vi "Host_timing_study_FPGA_check.vi"() -> ()   [LabVIEW 2019]
uses:
  <vilib>/Analysis/7linalg.llb/Eigenvalue and Vectors Output Option.ctl
  <vilib>/FPGAPlugInAG/PXIe-7915/niLvFpga_Open_PXIe-7915.vi
  <vilib>/rvi/interface/common/dynamic/niFpgaDynamicAddResources.vi
  <vilib>/Utility/error.llb/Error Cluster From Error Code.vi
  <vilib>/rvi/errors/niLvFpgaAdjustHostInterfaceError.vi
  <vilib>/FPGAPlugInAG/Dynamic/niLvFpga_Run_Dynamic.vi
  <vilib>/Analysis/baseanly.llb/Real Inverse Matrix.vi
  <vilib>/Analysis/Matrix/Numeric/Multiply/Multiply - RM,RM.vi
  <vilib>/Analysis/Matrix/Numeric/Add/Add - RM,RM.vi
  <vilib>/Analysis/Matrix/Numeric/Conversions/Matrix To Array - RM.vi
  <vilib>/Analysis/7linalg.llb/Real Eigenvalues and Vectors.vi
  <vilib>/FPGAPlugInAG/Dynamic/niLvFpga_Close_Dynamic.vi
  <vilib>/rvi/interface/nirviOpenFPGA/nirviOpenFPGA.xnode
  FPGA Bitfiles/Cholesky_SGL_19_nodes.lvbitx
  <vilib>/rvi/interface/nirviMethod/nirviMethod.xnode
  <vilib>/rvi/interface/nirviCloseFPGA/nirviCloseFPGA.xnode
  <vilib>/Analysis/NI_AALPro.lvlib
  <vilib>/Analysis/NI_AALBase.lvlib
  <vilib>/Analysis/Matrix/NI_Matrix.lvlib
  <vilib>/FPGAPlugInAG/Dynamic/niLvFpga_WriteFifo_Dynamic.vi
  <vilib>/rvi/errors/niLvFpgaMergeErrorWithErrorCode.vi
  <vilib>/FPGAPlugInAG/Dynamic/niLvFpga_ReadFifo_Dynamic.vi
panel:
  out "total run time (ms) 3":dbl
  out "total run time (ms) 2":dbl
  in  "stop":bool
  out "Eigenvalues":cdb[](array[numeric])
  out "total run time (ms)":dbl
  out "Frequencies":dbl[](array[numeric])
  out "K input":dbl[][](array[numeric])
  out "M input":dbl[][](array[numeric])
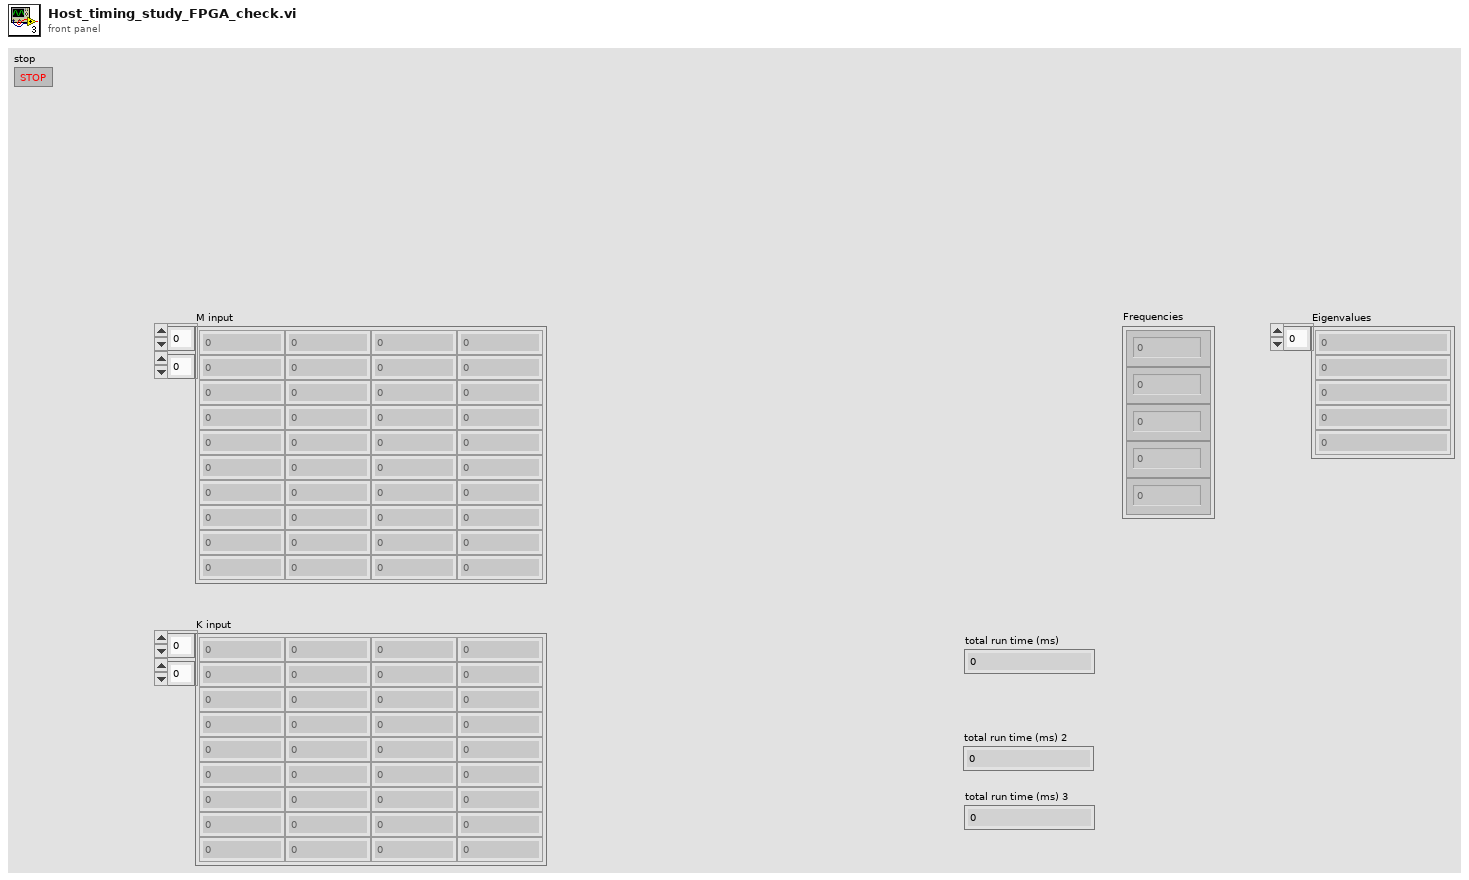
[diagram p1: front panel]
types:
  T1 = typedef "NI_AALPro.lvlib/Eigenvalue and Vectors Output Option.ctl" = i32
  T2 = typedef "NI_Matrix.lvlib/RealMatrix.ctl" = dbl[][]
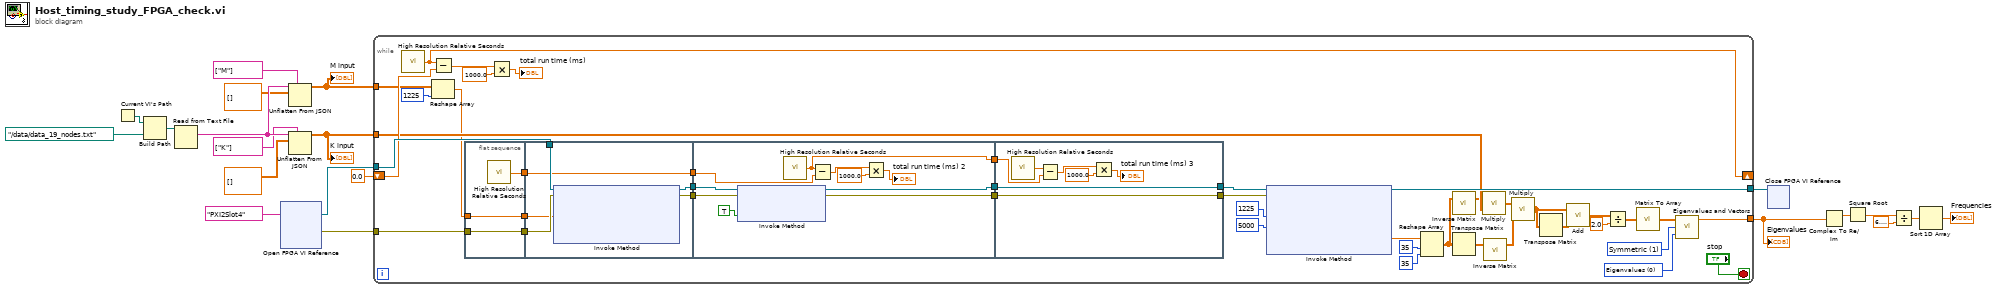
[diagram p0: block diagram]
diagram:
  n1 = Current VI's Path() -> (path=w15:path)
  n2 = Build Path(base path=w15, name or relative path=path "../data/data_19_nodes.txt") -> (appended path=w14:path)
  n3 = Read from Text File(file (use dialog)=w14) -> (text=w21:string)  [unwired: 3 in, 3 out]
  n4 = xnode "Open FPGA VI Reference"("resource name"=tag "PXI2Slot4") -> ("FPGA VI Reference Out"=w8:refnum<k20>, "error out"=w7:errorcluster)  [unwired: 1 in]
  n5 = Unflatten From JSON(path=string[] ["M"], JSON string=w21, type and defaults=dbl[][] []) -> (value=w3:dbl[][])  [unwired: 4 in, 1 out]
  "M input" <- w3
  n6 = Unflatten From JSON(path=string[] ["K"], JSON string=w21, type and defaults=dbl[][] []) -> (value=w4:dbl[][])  [unwired: 4 in, 1 out]
  "K input" <- w4
  n7 = while {
    tunnel: w8 -> [w64]
    tunnel: w7 -> [w63]
    tunnel: [w59] -> w5
    tunnel: w4 -> [w51]
    tunnel: w3 -> [w50]
    tunnel: [w57] -> w2
    shift-right: [w56] -> _
    shift-left: 0.0 ("relative seconds") -> [w55]
    stop <- "stop" stop-if-true
    w60 = T1 0 items=["Eigenvalues", "Eigenvalues & Vectors"] ("output option")
    w61 = 1 items=["General", "Symmetric"] ("matrix type")
    n8 = call <vilib>:"High Resolution Relative Seconds.vi"() -> ("relative seconds"=w56:dbl)
    n9 = Subtract(x=w56, y=w55) -> (x-y=w52:dbl)
    n10 = Reshape Array(w50, 1225 ("dimension size")) -> (w49:dbl[])
    n11 = flat-sequence {
      tunnel: w49 -> [w66]
      tunnel: w63 -> [w67]
      tunnel: [w67] -> w32
      tunnel: [w66] -> w31
      tunnel: [w65] -> w28
      tunnel: w64 -> [w73]
      tunnel: w32 -> [w72]
      tunnel: w31 -> [w71]
      tunnel: [w70] -> w30
      tunnel: [w69] -> w29
      tunnel: w28 -> [w68]
      tunnel: [w68] -> w27
      tunnel: w30 -> [w79]
      tunnel: w29 -> [w78]
      tunnel: w27 -> [w80]
      tunnel: [w76] -> w24
      tunnel: [w75] -> w23
      tunnel: [w74] -> w22
      tunnel: [w89] -> w25
      tunnel: [w90] -> w26
      tunnel: w24 -> [w90]
      tunnel: w23 -> [w89]
      tunnel: w22 -> [w84]
      frame #0 {
        n12 = call <vilib>:"High Resolution Relative Seconds.vi"() -> ("relative seconds"=w65:dbl)
      }
      frame #1 {
        n13 = xnode "Invoke Method"("FPGA VI Reference In"=w73, "error in"=w72, "Data"=w71) -> ("FPGA VI Reference Out"=w70:refnum<k20>, "error out"=w69:errorcluster)  [unwired: 1 in, 1 out]
      }
      frame #2 {
        n14 = xnode "Invoke Method"("FPGA VI Reference In"=w79, "error in"=w78, "Wait Until Done (F)"=TRUE) -> ("FPGA VI Reference Out"=w76:refnum<k20>, "error out"=w75:errorcluster)
        n15 = call <vilib>:"High Resolution Relative Seconds.vi"() -> ("relative seconds"=w74:dbl)
        n16 = Subtract(x=w74, y=w80) -> (x-y=w81:dbl)
        n17 = Multiply(x=w81, y=1000.0) -> (x*y=→"total run time (ms) 2":dbl)
      }
      frame #3 {
        n18 = call <vilib>:"High Resolution Relative Seconds.vi"() -> ("relative seconds"=w85:dbl)
        n19 = Subtract(x=w85, y=w84) -> (x-y=w86:dbl)
        n20 = Multiply(x=w86, y=1000.0) -> (x*y=→"total run time (ms) 3":dbl)
      }
    }
    n21 = Multiply(x=w52, y=1000.0) -> (x*y=→"total run time (ms)":dbl)
    n22 = xnode "Invoke Method"("FPGA VI Reference In"=w26, "error in"=w25, "Number of Elements"=u32 1225, "Timeout (ms)"=5000) -> ("FPGA VI Reference Out"=w57:refnum<k20>, "Data"=w36:sgl[])  [unwired: 2 out]
    n23 = Reshape Array(w36, 35 ("dimension size"), 35 ("dimension size")) -> (w35:sgl[][])
    n24 = call-poly <vilib>:"Inverse Matrix.vi"("Input Matrix"=w35) -> ("Inverse Matrix"=w45:T2)  [unwired: 1 in, 1 out]
    n25 = Transpose Matrix(1:w35) -> (0:w38:dbl[][])
    n26 = call-poly <vilib>:"Multiply.vi"("Real Matrix B"=w51, "Real Matrix A"=w45) -> ("A * B"=w43:T2)
    n27 = call-poly <vilib>:"Inverse Matrix.vi"("Input Matrix"=w38) -> ("Inverse Matrix"=w44:T2)  [unwired: 1 in, 1 out]
    n28 = call-poly <vilib>:"Multiply.vi"("Real Matrix B"=w44, "Real Matrix A"=w43) -> ("A * B"=w42:T2)
    n29 = Transpose Matrix(1:w42) -> (0:w41:T2)
    n30 = call-poly <vilib>:"Add.vi"("Real Matrix B"=w41, "Real Matrix A"=w42) -> ("A + B"=w39:T2)
    n31 = Divide(x=w39, y=2.0) -> (x/y=w33:T2)
    n32 = call-poly <vilib>:"Matrix To Array.vi"("Real Matrix"=w33) -> ("Real 2D Array"=w62:dbl[][])
    n33 = call-poly <vilib>:"Eigenvalues and Vectors.vi"("output option"=w60, "matrix type"=w61, "Input Matrix"=w62) -> ("Eigenvalues"=w59:cdb[])  [unwired: 2 out]
  }
  "Eigenvalues" <- w5
  n34 = xnode "Close FPGA VI Reference"("FPGA VI Reference In"=w2) -> ()  [unwired: 1 in, 1 out]
  n35 = Complex To Re/Im ("Complex To Cartesian.vi")(x + iy=w5) -> (x=w11:dbl[])  [unwired: 1 out]
  n36 = Square Root ("Square Root.vi")(x=w11) -> (sqrt(x)=w12:dbl[])
  n37 = Divide(x=w12, y=6.283185307179586) -> (x/y=w13:dbl[])
  n38 = Sort 1D Array(array=w13) -> (sorted array=→"Frequencies":dbl[])
